vi "UHR-Fleezers Control (host) - 12.7b.vi"() -> ()   [LabVIEW 2012] (continued)
                  tunnel: w664 -> [_ _ _ _ _ _ _ _ _ w685 _ _]
                  tunnel: w663 -> [_ _ _ _ _ _ _ _ _ w683 _ _]
                  frame #0 {
                    n399 = property on="Save ave N" class="DigNum (strict)"("Val(Sgnl)"=1.0 ("Value (Signaling)")) -> ()  [unwired: 2 in, 2 out]
                  }
                  frame #1 {
                    n400 = Wait (ms)(milliseconds to wait=u32 500) -> ()  [unwired: 1 out]
                  }
                  frame #2 {
                    n401 = property on="Trap Delta (MHz)" class="DigNum (strict)"("Val(Sgnl)"="Offset 2 Start (MHz)") -> ()  [unwired: 2 in, 2 out]
                    n402 = Replace Array Subset(array=u32[] [0] ("Index Values"), new element="Offset 2 Set", index=0) -> (w669:u32[])
                    n403 = property on="Saved AOD Raster Scan Parameter Sets" class="Arr (strict)"("Index Values"=w669) -> ()  [unwired: 2 in, 2 out]
                  }
                  frame #3 {
                    n404 = Wait (ms)(milliseconds to wait=u32 500) -> ()  [unwired: 1 out]
                  }
                  frame #4 {
                    n405 = property on="Load parameters" class="Bool (strict)"("Val(Sgnl)"=TRUE ("Value (Signaling)")) -> ()  [unwired: 2 in, 2 out]
                  }
                  frame #5 {
                    n406 = Wait (ms)(milliseconds to wait=u32 500) -> ()  [unwired: 1 out]
                  }
                  frame #6 {
                    n407 = property on="Trap Raster Scan" class="Bool (strict)"("Val(Sgnl)"=TRUE ("Value (Signaling)")) -> ()  [unwired: 2 in, 2 out]
                  }
                  frame #7 {
                    n408 = Wait (ms)(milliseconds to wait=u32 2000) -> ()  [unwired: 1 out]
                  }
                  frame #8 {
                    n409 = while {
                      stop <- w678 stop-if-true
                      n410 = local read "Raster Scanning..."() -> (w681:bool)
                      n411 = local read "Saving..."() -> (w679:bool)
                      n412 = Wait (ms)(milliseconds to wait=u32 100) -> ()  [unwired: 1 out]
                      n413 = Not(x=w679) -> (.not. x?=w677:bool)
                      n414 = Not(x=w681) -> (.not. x?=w680:bool)
                      n415 = And(x=w680, y=w677) -> (x .and. y?=w678:bool)
                    }
                  }
                  frame #9 {
                    n416 = property on="Trap Delta (MHz)" class="DigNum (strict)"("Val(Sgnl)"=w685) -> ()  [unwired: 2 in, 2 out]
                    n417 = property on="Saved AOD Raster Scan Parameter Sets" class="Arr (strict)"("Index Values"=u32[] [0]) -> ()  [unwired: 2 in, 2 out]
                    n418 = property on="Save ave N" class="DigNum (strict)"("Val(Sgnl)"=w683) -> ()  [unwired: 2 in, 2 out]
                  }
                  frame #10 {
                    n419 = Wait (ms)(milliseconds to wait=u32 500) -> ()  [unwired: 1 out]
                  }
                  frame #11 {
                    n420 = property on="Load parameters" class="Bool (strict)"("Val(Sgnl)"=TRUE ("Value (Signaling)")) -> ()  [unwired: 2 in, 2 out]
                  }
                }
              }
            }
          }
          frame #9 {
            n421 = property on="Read Cal" class="Bool (strict)"("Val(Sgnl)"=TRUE ("Value (Signaling)")) -> ()  [unwired: 2 in, 2 out]
          }
          frame #10 {
            n422 = Wait (ms)(milliseconds to wait=u32 1000) -> ()  [unwired: 1 out]
          }
          frame #11 {
            n423 = property on="Fish for Tether" class="Bool (strict)"("Val(Sgnl)"=TRUE ("Value (Signaling)")) -> ()  [unwired: 2 in, 2 out]
          }
        }
        n424 = local write "Cal/Data Acq. Spot"(FALSE ("Cal/Data Acq. Spot")) -> ()
      }
      event "Dump Beads": Value Change {
        n425 = event-data() -> ()  [unwired: 1 in, 5 out]
        n426 = flat-sequence {
          tunnel: ["Dump spot flow on?"] -> w691
          tunnel: [w702] -> w692
          tunnel: w691 -> [w702]
          tunnel: w695 -> [w707]
          tunnel: w694 -> [w706]
          tunnel: [w704] -> w693
          tunnel: w692 -> [w704]
          tunnel: w693 -> [w717]
          frame #0 {
            w696 = FALSE ("Value (Signaling)")
            n427 = local read "Saving..."() -> (w698:bool)
            n428 = local write "Dump Beads"(FALSE ("Dump Beads")) -> ()
            n429 = property on="Inject Pump 3" class="Bool (strict)"("Val(Sgnl)"=w696) -> ()  [unwired: 2 in, 2 out]
            n430 = property on="Inject Pump 1" class="Bool (strict)"("Val(Sgnl)"=w696) -> ()  [unwired: 2 in, 2 out]
            n431 = local write "Stop Saving"(w698) -> ()
          }
          frame #1 {
            w699 = FALSE ("Fl. Triggered...")
            n432 = case shown="True" "Dump spot flow on?" {
              frame False {
              }
              frame True {
                n433 = property on="Sample Channel\nFlow" class="Bool (strict)"("Val(Sgnl)"=TRUE ("Stage Moving")) -> ()  [unwired: 2 in, 2 out]
              }
            }
            n434 = local write "Fl. Triggered..."(w699) -> ()
            n435 = local write "Tether"(w699) -> ()
            n436 = property on="Green Laser ON" class="Bool (strict)"("Val(Sgnl)"=w699) -> ()  [unwired: 2 in, 2 out]
            n437 = property on="Trap Pos. FB ON" class="Bool (strict)"("Val(Sgnl)"=w699) -> ()  [unwired: 2 in, 2 out]
            n438 = property on="Trap Trig. Fl." class="Bool (strict)"("Val(Sgnl)"=w699) -> ()  [unwired: 2 in, 2 out]
            n439 = property on="Fl. Triggered..." class="Bool (strict)"("Val(Sgnl)"=w699) -> ()  [unwired: 2 in, 2 out]
            n440 = property on="Dip for Protein" class="Bool (strict)"("Val(Sgnl)"=w699) -> ()  [unwired: 2 in, 2 out]
            n441 = property on="Pause dwell" class="Bool (strict)"("Val(Sgnl)"=w699) -> ()  [unwired: 2 in, 2 out]
          }
          frame #2 {
            n442 = property on="Trap Pos. FB Offset Factor" class="DigNum (strict)"("Val(Sgnl)"=i64 0 ("Value (Signaling)")) -> ()  [unwired: 2 in, 2 out]
          }
          frame #3 {
            n443 = local read "Saved Stage Positions"() -> (w708:dbl[][])
            n444 = local write "Stage Moving"(TRUE ("Stage Moving")) -> ()
            n445 = Array Subset(array=w708, index (row)=3 ("index"), length (row)=1 ("length"), index (col)=1 ("index"), length (col)=3 ("length")) -> (w713:dbl[][])
            n446 = Reshape Array(w713, 3 ("dimension size")) -> (w711:dbl[])
            n447 = Array To Cluster(array=w711) -> (cluster=w710:cluster{"[0]":dbl, "[1]":dbl, "[2]":dbl})
            n448 = call "Set Stage Position.vi"("Position"=w710, "error in"=w706, "VISA resource name in"=w707) -> ()  [unwired: 3 out]
          }
          frame #4 {
            w718 = FALSE ("Value (Signaling)")
            n449 = case shown="True" w717 {
              frame False {
              }
              frame True {
                n450 = property on="Sample Channel\nFlow" class="Bool (strict)"("Val(Sgnl)"=FALSE ("Stage Moving")) -> ()  [unwired: 2 in, 2 out]
              }
            }
            n451 = property on="Trap 1 (ON/OFF)" class="Bool (strict)"("Val(Sgnl)"=w718) -> ()  [unwired: 2 in, 2 out]
            n452 = property on="Trap 2 (ON/OFF)" class="Bool (strict)"("Val(Sgnl)"=w718) -> ()  [unwired: 2 in, 2 out]
            n453 = call <vilib>:"Beep.vi"() -> ()  [unwired: 3 in, 9 out]
          }
          frame #5 {
            n454 = property on="Move Cap. 2 (ADig Top)" class="Bool (strict)"("Val(Sgnl)"=TRUE ("Value (Signaling)")) -> ()  [unwired: 2 in, 2 out]
            n455 = property on="Tab Control" class="TabCtl (strict)"("Val(Sgnl)"=T26."Status" ("Value (Signaling)")) -> ()  [unwired: 2 in, 2 out]
          }
        }
      }
      event "Dip for Protein": Value Change {
        n456 = event-data() -> ()  [unwired: 1 in, 5 out]
        n457 = case shown="True" "Dip for Protein" {
          tunnel: w724 -> [_ w726]
          tunnel: w723 -> [_ w725]
          frame False {
          }
          frame True {
            n458 = while {
              tunnel: w726 -> [w737]
              tunnel: w725 -> [w736]
              i -> [w731]
              stop <- w733 stop-if-true
              n459 = Increment(x=w731) -> (x+1=→"Dip #":i32)
              n460 = flat-sequence {
                tunnel: w736 -> [w748]
                tunnel: w737 -> [w749]
                tunnel: [w749] -> w741
                tunnel: [w748] -> w740
                tunnel: [w742] -> w727
                tunnel: [w754] -> w735
                tunnel: [w755] -> w734
                tunnel: w741 -> [w756]
                tunnel: w740 -> [w757]
                tunnel: [w752] -> w728
                tunnel: w727 -> [w752]
                tunnel: [w765] -> w739
                tunnel: w735 -> [w765]
                tunnel: [w764] -> w738
                tunnel: w734 -> [w764]
                tunnel: [w761] -> w732
                tunnel: [w760] -> w729
                tunnel: w728 -> [w760]
                tunnel: w738 -> [w785]
                tunnel: w739 -> [w786]
                tunnel: w732 -> [w787]
                tunnel: w729 -> [w784]
                tunnel: [w843] -> w733
                frame #0 {
                  n461 = local read "Trap Pos. FB ON"() -> (w742:bool)
                  n462 = Compound Arithmetic op=AND("Flow ON\nduring dip?", "FB OFF when \nflow ON", w742) -> (w743:bool)
                  n463 = case shown="True" "Move trap \nbefore dip move?" {
                    frame False {
                    }
                    frame True {
                      n464 = property on="Trap Delta (MHz)" class="DigNum (strict)"("Val(Sgnl)"="Dipping Delta (MHz)") -> ()  [unwired: 2 in, 2 out]
                    }
                  }
                  n465 = property on="Green Laser ON" class="Bool (strict)"("Val(Sgnl)"="Green ON\nbefore dip?") -> ()  [unwired: 2 in, 2 out]
                  n466 = property on="Sample Channel\nFlow" class="Bool (strict)"("Val(Sgnl)"="Flow ON\nduring dip?") -> ()  [unwired: 2 in, 2 out]
                  n467 = case shown="True" w743 {
                    frame False {
                    }
                    frame True {
                      n468 = property on="Trap Pos. FB ON" class="Bool (strict)"("Val(Sgnl)"=FALSE ("Value (Signaling)")) -> ()  [unwired: 2 in, 2 out]
                    }
                  }
                }
                frame #1 {
                  n469 = local read "Saved Stage Positions"() -> (w759:dbl[][])
                  n470 = local write "Cancel dwell"(FALSE ("Cancel dwell")) -> ()
                  n471 = call "move to saved stage position.vi"("error in"=w757, "Stage VISA resource name in"=w756, "Position"="Dip Stage \nPosition", "Saved Stage Positions"=w759) -> ("VISA resource name out"=w754:refnum<visa-resource-name>, "error out"=w755:errorcluster)
                }
                frame #2 {
                  n472 = node-c288() -> (w763:T23)  [unwired: 4 in]
                  n473 = timed-loop {
                    timing: w763 -> [_]
                    timing-out: [_] -> w762
                    tunnel: [w769] -> w761
                    i -> [w766]
                    stop <- w770 stop-if-true
                    n474 = node-c288() -> ()  [unwired: 1 in, 1 out]
                    n475 = Greater Or Equal?(x=w766, y="Dip Duration (s)") -> (x >= y?=w778:bool)
                    n476 = local read "Dip for Protein"() -> (w771:bool)
                    n477 = local read "Dump Beads"() -> (w768:bool)
                    n478 = local read "Cancel dwell"() -> (w777:bool)
                    n479 = local read "Pause dwell"() -> (w774:bool)
                    n480 = Not(x=w771) -> (.not. x?=w776:bool)
                    n481 = Compound Arithmetic op=OR(w777, w778, w776) -> (w775:bool)
                    n482 = Select(t=FALSE, s=w774, f=w775) -> (s? t:f=w772:bool)
                    n483 = Not(x=w768) -> (.not. x?=w767:bool)
                    n484 = node-c288() -> ()  [unwired: 1 in, 1 out]
                    n485 = And(x=w771, y=w767) -> (x .and. y?=w769:bool)
                    n486 = Or(x=w772, y=w768) -> (x .or. y?=w770:bool)
                    "Dip Time (s)" <- w766
                  }
                  n487 = node-c288(w762) -> ()  [unwired: 1 out]
                }
                frame #3 {
                  n488 = case shown="True" w787 {
                    tunnel: w786 -> [_ w792]
                    tunnel: w785 -> [_ w791]
                    tunnel: w784 -> [_ w788]
                    frame False {
                    }
                    frame True {
                      n489 = flat-sequence {
                        tunnel: w791 -> [w796]
                        tunnel: w792 -> [w797]
                        tunnel: [w797] -> w790
                        tunnel: [w796] -> w789
                        tunnel: w788 -> [w793]
                        tunnel: w790 -> [w807]
                        tunnel: w789 -> [w806]
                        tunnel: w788 -> [w815]
                        frame #0 {
                          n490 = local read "Sample Channel\nFlow"() -> (w795:bool)
                          n491 = case shown="True" w795 {
                            tunnel: "Flow ON \nduring return\nfrom dip?" -> [w798 w801]
                            tunnel: w793 -> [_ w800]
                            frame False {
                              n492 = case shown="True" w798 {
                                frame False {
                                }
                                frame True {
                                n493 = property on="Sample Channel\nFlow" class="Bool (strict)"("Val(Sgnl)"=TRUE ("Value (Signaling)")) -> ()  [unwired: 2 in, 2 out]
                                }
                              }
                            }
                            frame True {
                              n494 = case shown="False" w801 {
                                tunnel: w800 -> [w802 _]
                                frame False {
                                n495 = property on="Trap Pos. FB ON" class="Bool (strict)"("Val(Sgnl)"=w802) -> ()  [unwired: 2 in, 2 out]
                                n496 = property on="Sample Channel\nFlow" class="Bool (strict)"("Val(Sgnl)"=FALSE ("Value (Signaling)")) -> ()  [unwired: 2 in, 2 out]
                                }
                                frame True {
                                }
                              }
                            }
                          }
                        }
                        frame #1 {
                          # "For turning on green laser before stage reaches lower spot"
                          n497 = case shown="True" "Green ON\nafter start\nreturn?" {
                            frame False {
                            }
                            frame True {
                              n498 = flat-sequence {
                                frame #0 {
                                n499 = Multiply(x="Green delay after \nstart return (s)", y=1000.0) -> (x*y=w812:dbl)
                                n500 = Wait (ms)(milliseconds to wait=w812) -> ()  [unwired: 1 out]
                                }
                                frame #1 {
                                n501 = property on="Green Laser ON" class="Bool (strict)"("Val(Sgnl)"=TRUE ("Value (Signaling)")) -> ()  [unwired: 2 in, 2 out]
                                }
                              }
                            }
                          }
                          n502 = local read "Saved Stage Positions"() -> (w810:dbl[][])
                          n503 = local write "Cancel dwell"(FALSE ("Cancel dwell")) -> ()
                          n504 = call "move to saved stage position.vi"("error in"=w806, "Stage VISA resource name in"=w807, "Position"="Return Stage \nPosition", "Saved Stage Positions"=w810) -> ("error out"=w808:errorcluster)  [unwired: 1 out]
                          n505 = local write "Stage Control Serial Error"(w808) -> ()
                        }
                        frame #2 {
                          n506 = property on="Trap Pos. FB ON" class="Bool (strict)"("Val(Sgnl)"=w815) -> ()  [unwired: 2 in, 2 out]
                          n507 = case shown="True" "Green ON \nafter return?" {
                            frame False {
                            }
                            frame True {
                              n508 = property on="Green Laser ON" class="Bool (strict)"("Val(Sgnl)"=TRUE ("Value (Signaling)")) -> ()  [unwired: 2 in, 2 out]
                            }
                          }
                          n509 = case shown="True" "Move trap after return?" {
                            frame False {
                            }
                            frame True {
                              n510 = property on="Trap Delta (MHz)" class="DigNum (strict)"("Val(Sgnl)"="Dip Trap Delta 2 (MHz)") -> ()  [unwired: 2 in, 2 out]
                            }
                          }
                          n511 = case shown="True" "Save data after return?" {
                            frame False {
                            }
                            frame True {
                              n512 = property on="Start Saving" class="Bool (strict)"("Val(Sgnl)"=TRUE ("Value (Signaling)")) -> ()  [unwired: 2 in, 2 out]
                            }
                          }
                          n513 = property on="Sample Channel\nFlow" class="Bool (strict)"("Val(Sgnl)"="Flow ON\nduring daq?") -> ()  [unwired: 2 in, 2 out]
                        }
                        frame #3 {
                          n514 = node-c288() -> (w824:T23)  [unwired: 4 in]
                          n515 = timed-loop {
                            timing: w824 -> [_]
                            timing-out: [_] -> w823
                            i -> [w825]
                            stop <- w827 stop-if-true
                            n516 = node-c288() -> ()  [unwired: 1 in, 1 out]
                            n517 = local read "Dump Beads"() -> (w826:bool)
                            n518 = Greater Or Equal?(x=w825, y="Dwell Duration (s)") -> (x >= y?=w832:bool)
                            n519 = local read "Dip for Protein"() -> (w829:bool)
                            n520 = Not(x=w829) -> (.not. x?=w828:bool)
                            n521 = Compound Arithmetic op=OR(w832, "Cancel dwell", w828) -> (w831:bool)
                            n522 = node-c288() -> ()  [unwired: 1 in, 1 out]
                            n523 = Select(t=FALSE, s="Pause dwell", f=w831) -> (s? t:f=w834:bool)
                            n524 = Or(x=w834, y=w826) -> (x .or. y?=w827:bool)
                            "Dwell Time (s)" <- w825
                          }
                          n525 = node-c288(w823) -> ()  [unwired: 1 out]
                        }
                      }
                    }
                  }
                }
                frame #4 {
                  n526 = local read "Dip for Protein"() -> (w844:bool)
                  n527 = local read "Dump Beads"() -> (w841:bool)
                  n528 = local write "Cancel dwell"(FALSE ("Cancel dwell")) -> ()
                  n529 = Not(x=w844) -> (.not. x?=w845:bool)
                  n530 = Not(x="Cont. Repeat Dipping?") -> (.not. x?=w847:bool)
                  n531 = Compound Arithmetic op=OR(w845, w847, w841) -> (w843:bool)
                }
              }
            }
          }
        }
      }
      event "Profile": Value Change {
        n532 = event-data() -> ()  [unwired: 1 in, 5 out]
        n533 = flat-sequence {
          tunnel: w856 -> [w859]
          tunnel: w855 -> [w867]
          tunnel: [w861] -> w854
          tunnel: [w860] -> w853
          tunnel: [w858] -> w851
          tunnel: [w857] -> w848
          tunnel: w854 -> [w874]
          tunnel: w853 -> [w873]
          tunnel: [w871] -> w852
          tunnel: w851 -> [w872]
          tunnel: [w870] -> w850
          tunnel: [w869] -> w849
          tunnel: w848 -> [w869]
          tunnel: w852 -> [w878]
          tunnel: w850 -> [w877]
          tunnel: w849 -> [w876]
          frame #0 {
            n534 = call "Read Stage Position.vi"("error in"=w867, "VISA resource name in"=w859) -> ("Current Position"=w857:cluster{dbl, dbl, dbl}, "error out"=w860:errorcluster, "VISA resource name out"=w858:refnum<visa-resource-name>)  [unwired: 1 out]
            "Current Position" <- w857
            n535 = local write "Stage Control Serial Error"(w860) -> ()
            n536 = Unbundle(w857) -> (w864:dbl, w866:dbl, w862:dbl)
            n537 = Add(x=w866, y="Y change (mm)") -> (x+y=w863:dbl)
            n538 = Bundle(w864, w863, w862) -> (w861:cluster{dbl, dbl, dbl})  [unwired: 1 in]
          }
          frame #1 {
            # "move to new position and start saving"
            n539 = local write "Stage Moving"(TRUE ("Stage Moving")) -> ()
            n540 = local write "Start Saving"(TRUE ("Start Saving")) -> ()
            n541 = call "Set Stage Position.vi"("Position"=w874, "error in"=w873, "VISA resource name in"=w872) -> ("error out"=w870:errorcluster, "VISA resource name out"=w871:refnum<visa-resource-name>)  [unwired: 1 out]
          }
          frame #2 {
            # "go back to start"
            n542 = call "Set Stage Position.vi"("Position"=w876, "error in"=w877, "VISA resource name in"=w878) -> ()  [unwired: 3 out]
          }
          frame #3 {
            # "stop saving"
            n543 = local write "Stop Saving"(TRUE ("Stop Saving")) -> ()
            n544 = local write "Stage Moving"(FALSE ("Stage Moving")) -> ()
          }
        }
      }
      event "Move to Position 1", "Move to Position 2", "Move to Position 3", "Move to Position 4", "Move to Position 5", "Lower Ch. Cap.": Value Change {
        n545 = event-data() -> ()  [unwired: 1 in, 5 out]
        n546 = Or(x="Move to Position 5", y="Lower Ch. Cap.") -> (x .or. y?=w884:bool)
        n547 = Build Array("Move to Position 1", "Move to Position 2", "Move to Position 3", "Move to Position 4", w884) -> (w887:bool[])
        n548 = Boolean Array To Number(Boolean array=w887) -> (number=w886:u32)
        n549 = Logarithm Base 2(1:w886) -> (0:w885:dbl)
        n550 = flat-sequence {
          tunnel: w885 -> [w896]
          tunnel: w882 -> [w894]
          tunnel: w881 -> [w893]
          frame #0 {
            n551 = local read "Saved Stage Positions"() -> (w904:dbl[][])
            n552 = Array Subset(array=w904, index (row)=w896, length (row)=1 ("length"), index (col)=1 ("index"), length (col)=3 ("length")) -> (w901:dbl[][])
            n553 = Reshape Array(w901, 3 ("dimension size")) -> (w899:dbl[])
            n554 = Array To Cluster(array=w899) -> (cluster=w898:cluster{"[0]":dbl, "[1]":dbl, "[2]":dbl})
            n555 = call "Set Stage Position.vi"("Position"=w898, "error in"=w893, "VISA resource name in"=w894) -> ("error out"=w897:errorcluster)  [unwired: 2 out]
            n556 = local write "Stage Moving"(TRUE ("Stage Moving")) -> ()
            n557 = local write "Stage Control Serial Error"(w897) -> ()
          }
          frame #1 {
            n558 = local write "Stage Moving"(FALSE ("Stage Moving")) -> ()
            n559 = call <vilib>:"Beep.vi"() -> ()  [unwired: 3 in, 9 out]
          }
        }
      }
      event "Got ADig bead": Value Change {
        n560 = event-data() -> ()  [unwired: 1 in, 5 out]
        n561 = flat-sequence {
          frame #0 {
            n562 = local read "Cap 1 Samp Flow ON"() -> (w908:bool)
            n563 = case shown="True" w908 {
              frame False {
              }
              frame True {
                n564 = property on="Sample Channel\nFlow" class="Bool (strict)"("Val(Sgnl)"=TRUE ("Value (Signaling)")) -> ()  [unwired: 2 in, 2 out]
              }
            }
          }
          frame #1 {
            n565 = property on="Inject Pump 3" class="Bool (strict)"("Val(Sgnl)"=FALSE ("Value (Signaling)")) -> ()  [unwired: 2 in, 2 out]
          }
          frame #2 {
            n566 = property on="Move Cap. 1 (DNA Bottom)" class="Bool (strict)"("Val(Sgnl)"=TRUE ("Value (Signaling)")) -> ()  [unwired: 2 in, 2 out]
          }
        }
      }
      event "Force FB Data\nScript": Value Change {
        n567 = event-data() -> ()  [unwired: 1 in, 5 out]
        n568 = flat-sequence {
          tunnel: w917 -> [w921]
          tunnel: w918 -> [w922]
          tunnel: [w922] -> w913
          tunnel: [w921] -> w912
          tunnel: w913 -> [w925]
          tunnel: w912 -> [w924]
          tunnel: ["Trap Trig Fl."] -> w914
          tunnel: [w950] -> w915
          tunnel: w914 -> [w950]
          tunnel: [w954] -> w916
          tunnel: w915 -> [w954]
          tunnel: w916 -> [w956]
          frame #0 {
            n569 = property on="Trap Delta (MHz)" class="DigNum (strict)"("Val(Sgnl)"="Trap Delta Before Moving") -> ()  [unwired: 2 in, 2 out]
          }
          frame #1 {
            n570 = local read "Saved Stage Positions"() -> (w927:dbl[][])
            n571 = local write "FB Trap Pos Offset"(0.0 ("FB Trap Pos Offset")) -> ()
            n572 = property on="Trap Pos. FB Offset Factor" class="DigNum (strict)"("Val(Sgnl)"=i64 0 ("Value (Signaling)")) -> ()  [unwired: 2 in, 2 out]
            n573 = local write "Stage Moving"(TRUE ("Stage Moving")) -> ()
            n574 = call "move to saved stage position.vi"("error in"=w924, "Stage VISA resource name in"=w925, "Position"="Stage Position To Establish FB", "Saved Stage Positions"=w927) -> ("error out"=w923:errorcluster)  [unwired: 1 out]
            n575 = local write "Stage Control Serial Error"(w923) -> ()
          }
          frame #2 {
            n576 = call <vilib>:"Beep.vi"() -> ()  [unwired: 3 in, 9 out]
            n577 = Multiply(x="Wait (s)", y=u32 1000 ("milliseconds to wait")) -> (x*y=w934:u32)
            n578 = property on="Trap Delta (MHz)" class="DigNum (strict)"("Val(Sgnl)"="Starting \nTrap Delta (MHz)") -> ()  [unwired: 2 in, 2 out]
            n579 = local write "Stage Moving"(FALSE ("Stage Moving")) -> ()
            n580 = Wait (ms)(milliseconds to wait=w934) -> ()  [unwired: 1 out]
            n581 = property on="Tab Control 2" class="TabCtl (strict)"("Val(Sgnl)"=T6."Feedback on Trap Position" ("Value (Signaling)")) -> ()  [unwired: 2 in, 2 out]
            n582 = property on="Tab Control" class="TabCtl (strict)"("Val(Sgnl)"=T27."Trap Control (RF)" ("Value (Signaling)")) -> ()  [unwired: 2 in, 2 out]
          }
          frame #3 {
            n583 = property on="Set Reading to\nSetpoint" class="Bool (strict)"("Val(Sgnl)"=TRUE ("Value (Signaling)")) -> ()  [unwired: 2 in, 2 out]
            n584 = Wait (ms)(milliseconds to wait=u32 500) -> ()  [unwired: 1 out]
          }
          frame #4 {
            n585 = property on="Trap Pos. FB ON" class="Bool (strict)"("Val(Sgnl)"=TRUE ("Value (Signaling)")) -> ()  [unwired: 2 in, 2 out]
            n586 = Wait (ms)(milliseconds to wait=u32 250) -> ()  [unwired: 1 out]
          }
          frame #5 {
            n587 = case shown="False" "Trap Trig Fl." {
              frame False {
                n588 = case shown="True" "Green ON after FB ON?" {
                  selector: "Green ON after FB ON?" -> [_ w949]
                  frame False {
                  }
                  frame True {
                    n589 = property on="Green Laser ON" class="Bool (strict)"("Val(Sgnl)"=w949) -> ()  [unwired: 2 in, 2 out]
                  }
                }
              }
              frame True {
              }
            }
            n590 = case shown="True" "Remove Action Offset" {
              tunnel: TRUE ("Value (Signaling)") -> [w946 w947]
              frame False {
                n591 = property on="Remove Unwinding Offset" class="Bool (strict)"("Val(Sgnl)"=w946) -> ()  [unwired: 2 in, 2 out]
              }
              frame True {
                n592 = property on="Remove Action Offset" class="Bool (strict)"("Val(Sgnl)"=w947) -> ()  [unwired: 2 in, 2 out]
              }
            }
            n593 = Wait (ms)(milliseconds to wait=u32 250) -> ()  [unwired: 1 out]
          }
          frame #6 {
            n594 = property on="Start Saving" class="Bool (strict)"("Val(Sgnl)"=TRUE ("Value (Signaling)")) -> ()  [unwired: 2 in, 2 out]
            n595 = Wait (ms)(milliseconds to wait=u32 5000) -> ()  [unwired: 1 out]
          }
          frame #7 {
            w953 = TRUE ("Value (Signaling)")
            n596 = property on="Rem fb disp offset" class="Bool (strict)"("Val(Sgnl)"=w953) -> ()  [unwired: 2 in, 2 out]
            n597 = property on="Remove Offset" class="Bool (strict)"("Val(Sgnl)"=w953) -> ()  [unwired: 2 in, 2 out]
            n598 = Wait (ms)(milliseconds to wait=u32 100) -> ()  [unwired: 1 out]
          }
          frame #8 {
            n599 = case shown="True" w956 {
              frame False {
              }
              frame True {
                n600 = local write "Trap Trig. Fl."(TRUE ("Value (Signaling)")) -> ()
              }
            }
          }
          frame #9 {
            n601 = case shown="True" "Start dipping after?" {
              frame False {
              }
              frame True {
                n602 = flat-sequence {
                  frame #0 {
                    n603 = Multiply(x="Delay before dipping (s)", y=1000.0) -> (x*y=w960:dbl)
                    n604 = Wait (ms)(milliseconds to wait=w960) -> ()  [unwired: 1 out]
                  }
                  frame #1 {
                    n605 = property on="Dip for Protein" class="Bool (strict)"("Val(Sgnl)"=TRUE ("Value (Signaling)")) -> ()  [unwired: 2 in, 2 out]
                    n606 = local write "Scripts"(T1."Dipping" ("Scripts")) -> ()
                  }
                }
              }
            }
          }
        }
      }
      event "Fixed Traps Data\nScript": Value Change {
        n607 = event-data() -> ()  [unwired: 1 in, 5 out]
        n608 = flat-sequence {
          frame #0 {
            n609 = case shown="True" "Green ON" {
              frame False {
              }
              frame True {
                n610 = property on="Green Laser ON" class="Bool (strict)"("Val(Sgnl)"=TRUE) -> ()  [unwired: 2 in, 2 out]
              }
            }
            n611 = local write "Offset (nm)"(0.0 ("Offset (nm)")) -> ()
            n612 = property on="Sample Channel\nFlow" class="Bool (strict)"("Val(Sgnl)"=FALSE ("Value (Signaling)")) -> ()  [unwired: 2 in, 2 out]
            n613 = property on="Trap Delta (MHz)" class="DigNum (strict)"("Val(Sgnl)"="Fixed Traps Trap Delta (MHz)") -> ()  [unwired: 2 in, 2 out]
          }
          frame #1 {
            n614 = Wait (ms)(milliseconds to wait=u32 1000) -> ()  [unwired: 1 out]
          }
          frame #2 {
            n615 = local write "Start Saving"(TRUE ("Start Saving")) -> ()
          }
          frame #3 {
            n616 = local read "Bead Sep. Int. Time (s)"() -> (w971:dbl)
            n617 = Multiply(x=w971, y=1000.0) -> (x*y=w973:dbl)
            n618 = Wait (ms)(milliseconds to wait=w973) -> ()  [unwired: 1 out]
          }
          frame #4 {
            n619 = property on="Remove Offset" class="Bool (strict)"("Val(Sgnl)"=TRUE ("Value (Signaling)")) -> ()  [unwired: 2 in, 2 out]
          }
          frame #5 {
            n620 = property on="Dip for Protein" class="Bool (strict)"("Val(Sgnl)"="Start dipping after?") -> ()  [unwired: 2 in, 2 out]
          }
        }
      }
      event "Got DNA bead": Value Change {
        n621 = event-data() -> ()  [unwired: 1 in, 5 out]
        n622 = flat-sequence {
          frame #0 {
            n623 = local read "Daq spot flow on"() -> (w978:bool)
            n624 = case shown="True" w978 {
              frame False {
              }
              frame True {
                n625 = property on="Sample Channel\nFlow" class="Bool (strict)"("Val(Sgnl)"=TRUE ("Value (Signaling)")) -> ()  [unwired: 2 in, 2 out]
              }
            }
            n626 = property on="Got DNA bead" class="Bool"("Key Focus"=FALSE) -> ()  [unwired: 2 in, 2 out]
          }
          frame #1 {
            n627 = property on="Inject Pump 1" class="Bool (strict)"("Val(Sgnl)"=FALSE ("Value (Signaling)")) -> ()  [unwired: 2 in, 2 out]
          }
          frame #2 {
            n628 = property on="Cal/Data Acq. Spot" class="Bool (strict)"("Val(Sgnl)"=TRUE ("Value (Signaling)")) -> ()  [unwired: 2 in, 2 out]
          }
        }
      }
      event "Take Stepping Data": Value Change {
        n629 = event-data() -> ()  [unwired: 1 in, 5 out]
        n630 = local read "Save ave N"() -> (w990:dbl)
        n631 = flat-sequence {
          tunnel: w990 -> [w992]
          tunnel: [w992] -> w985
          tunnel: [w994] -> w986
          tunnel: w985 -> [w994]
          tunnel: [w996] -> w987
          tunnel: w986 -> [w996]
          tunnel: [w999] -> w988
          tunnel: w987 -> [w999]
          tunnel: [w1001] -> w989
          tunnel: w988 -> [w1001]
          tunnel: [w1003] -> w983
          tunnel: w989 -> [w1003]
          tunnel: w983 -> [w1006]
          tunnel: [w1006] -> w982
          tunnel: w982 -> [w1007]
          tunnel: [w1007] -> w984
          tunnel: w984 -> [w1013]
          frame #0 {
            n632 = property on="Save ave N" class="DigNum (strict)"("Val(Sgnl)"="Save ave factor") -> ()  [unwired: 2 in, 2 out]
          }
          frame #1 {
            n633 = Wait (ms)(milliseconds to wait=u32 100) -> ()  [unwired: 1 out]
          }
          frame #2 {
            n634 = local read "Offset 2 Start (MHz)"() -> (w998:dbl)
            n635 = property on="Saved AOD Raster Scan Parameter Sets" class="Arr (strict)"("Index Values"=u32[] [2]) -> ()  [unwired: 2 in, 2 out]
            n636 = property on="Trap Delta (MHz)" class="DigNum (strict)"("Val(Sgnl)"=w998) -> ()  [unwired: 2 in, 2 out]
          }
          frame #3 {
            n637 = property on="Load parameters" class="Bool (strict)"("Val(Sgnl)"=TRUE ("Value (Signaling)")) -> ()  [unwired: 2 in, 2 out]
          }
          frame #4 {
            n638 = Wait (ms)(milliseconds to wait=u32 100) -> ()  [unwired: 1 out]
          }
          frame #5 {
            n639 = property on="Trap Raster Scan" class="Bool (strict)"("Val(Sgnl)"=TRUE ("Value (Signaling)")) -> ()  [unwired: 2 in, 2 out]
          }
          frame #6 {
            n640 = Wait (ms)(milliseconds to wait=u32 1000) -> ()  [unwired: 1 out]
          }
          frame #7 {
            n641 = while {
              stop <- w1010 stop-if-true
              n642 = local read "Raster Scanning..."() -> (w1012:bool)
              n643 = local read "Saving..."() -> (w1011:bool)
              n644 = Not(x=w1011) -> (.not. x?=w1008:bool)
              n645 = Not(x=w1012) -> (.not. x?=w1009:bool)
              n646 = And(x=w1009, y=w1008) -> (x .and. y?=w1010:bool)
            }
          }
          frame #8 {
            n647 = property on="Save ave N" class="DigNum (strict)"("Val(Sgnl)"=w1013) -> ()  [unwired: 2 in, 2 out]
          }
        }
      }
      event "Step Size (nm)": Value Change {
        n648 = event-data() -> ()  [unwired: 1 in, 5 out]
        n649 = flat-sequence {
          frame #0 {
            n650 = property on="Saved AOD Raster Scan Parameter Sets" class="Arr (strict)"("Index Values"=u32[] [1]) -> ()  [unwired: 2 in, 2 out]
          }
          frame #1 {
            n651 = Multiply(x="N Steps", y="Step Size (nm)") -> (x*y=w1015:dbl)
            n652 = property on="Scan Speed AOD (nm/s) 2" class="DigNum (strict)"("Value"="Step Size (nm)") -> ()  [unwired: 2 in, 2 out]
            n653 = property on="Step Size AOD (nm) 2" class="DigNum (strict)"("Value"="Step Size (nm)") -> ()  [unwired: 2 in, 2 out]
            n654 = property on="Scan Range AOD (nm) 2" class="DigNum (strict)"("Value"=w1015) -> ()  [unwired: 2 in, 2 out]
          }
        }
      }
      event "Take Detection Laser\nImage": Value Change {
        n655 = event-data() -> ()  [unwired: 1 in, 5 out]
        n656 = flat-sequence {
          tunnel: [w1043] -> w1033
          tunnel: [w1042] -> w1026
          tunnel: [w1041] -> w1018
          tunnel: [w1046] -> w1034
          tunnel: w1033 -> [w1046]
          tunnel: [w1045] -> w1027
          tunnel: w1026 -> [w1045]
          tunnel: [w1044] -> w1019
          tunnel: w1018 -> [w1044]
          tunnel: [w1050] -> w1035
          tunnel: w1034 -> [w1050]
          tunnel: [w1049] -> w1028
          tunnel: w1027 -> [w1049]
          tunnel: [w1048] -> w1020
          tunnel: w1019 -> [w1048]
          tunnel: [w1056] -> w1036
          tunnel: w1035 -> [w1056]
          tunnel: [w1055] -> w1029
          tunnel: w1028 -> [w1055]
          tunnel: [w1054] -> w1021
          tunnel: w1020 -> [w1054]
          tunnel: [w1060] -> w1037
          tunnel: w1036 -> [w1060]
          tunnel: [w1059] -> w1030
          tunnel: w1029 -> [w1059]
          tunnel: [w1058] -> w1022
          tunnel: w1021 -> [w1058]
          tunnel: [w1064] -> w1038
          tunnel: w1037 -> [w1064]
          tunnel: [w1063] -> w1031
          tunnel: w1030 -> [w1063]
          tunnel: [w1062] -> w1023
          tunnel: w1022 -> [w1062]
          tunnel: [w1068] -> w1039
          tunnel: w1038 -> [w1068]
          tunnel: [w1067] -> w1032
          tunnel: w1031 -> [w1067]
          tunnel: [w1066] -> w1024
          tunnel: w1023 -> [w1066]
          tunnel: w1039 -> [w1074]
          tunnel: w1032 -> [w1073]
          tunnel: [w1071] -> w1025
          tunnel: w1024 -> [w1071]
          tunnel: w1025 -> [w1075]
          frame #0 {
            n657 = local read "Laser interlacing mode"() -> (w1042:enum32{"Laser ON", "Laser OFF", "Interlace"})
            n658 = local read "Green FB On/Off"() -> (w1041:bool)
            n659 = local read "Green Laser ON"() -> (w1043:bool)
          }
          frame #1 {
            n660 = property on="Green FB On/Off" class="Bool (strict)"("Val(Sgnl)"=FALSE ("Value (Signaling)")) -> ()  [unwired: 2 in, 2 out]
          }
          frame #2 {
            n661 = property on="Green Laser ON" class="Bool (strict)"("Val(Sgnl)"=TRUE ("Value (Signaling)")) -> ()  [unwired: 2 in, 2 out]
            n662 = property on="Flip Green Filter" class="Bool (strict)"("Val(Sgnl)"=TRUE ("Value (Signaling)")) -> ()  [unwired: 2 in, 2 out]
            n663 = property on="Laser interlacing mode" class="RadioBtnsControl (strict)"("Val(Sgnl)"=enum32{"Laser ON", "Laser OFF", "Interlace"}."Laser ON" ("Value (Signaling)")) -> ()  [unwired: 2 in, 2 out]
          }
          frame #3 {
            n664 = Wait (ms)(milliseconds to wait=u32 500) -> ()  [unwired: 1 out]
          }
          frame #4 {
            n665 = property on="Confocal Image" class="Bool (strict)"("Val(Sgnl)"=TRUE ("Value (Signaling)")) -> ()  [unwired: 2 in, 2 out]
          }
          frame #5 {
            n666 = Wait (ms)(milliseconds to wait=u32 2000) -> ()  [unwired: 1 out]
          }
          frame #6 {
            n667 = while {
              stop <- w1069 stop-if-true
              n668 = local read "Saving..."() -> (w1070:bool)
              n669 = Not(x=w1070) -> (.not. x?=w1069:bool)
            }
          }
          frame #7 {
            n670 = property on="Flip Green Filter" class="Bool (strict)"("Val(Sgnl)"=TRUE ("Value (Signaling)")) -> ()  [unwired: 2 in, 2 out]
            n671 = property on="Green Laser ON" class="Bool (strict)"("Val(Sgnl)"=w1074) -> ()  [unwired: 2 in, 2 out]
            n672 = property on="Laser interlacing mode" class="RadioBtnsControl (strict)"("Val(Sgnl)"=w1073) -> ()  [unwired: 2 in, 2 out]
          }
          frame #8 {
            n673 = property on="Green FB On/Off" class="Bool (strict)"("Val(Sgnl)"=w1075) -> ()  [unwired: 2 in, 2 out]
          }
        }
      }
      event "Move in a Circle": Value Change {
        # "converting distance (d) to angle (a)\na=arcsin(d/2r)"
        # "radius"
        # "radius"
        # "T1 Y"
        # "T1 X"
        n674 = event-data() -> ()  [unwired: 1 in, 5 out]
        n675 = local read "BD 2 Frequency 1 (MHz)"() -> (w1080:dbl)
        n676 = local read "BD 1 Frequency 2 (MHz)"() -> (w1079:dbl)
        n677 = local read "BD 2 Frequency 2 (MHz)"() -> (w1078:dbl)
        n678 = local read "BD 1 Frequency 1 (MHz)"() -> (w1081:dbl)
        n679 = Subtract(x=w1080, y="Center Y Frequency (MHz)") -> (x-y=w1090:dbl)
        n680 = Absolute Value(x=w1090) -> (abs(x)=w1086:dbl)
        n681 = Multiply(x=w1086, y=2) -> (x*y=w1085:dbl)
        n682 = Divide(x="2D Motion Trap Separation (MHz)", y=w1085) -> (x/y=w1083:dbl)
        n683 = Inverse Sine(1:w1083) -> (0:w1087:dbl)
        n684 = Multiply(x=w1087, y=2) -> (x*y=w1082:dbl)
        n685 = node-c288() -> (w1092:T23)  [unwired: 4 in]
        n686 = timed-loop {
          tunnel: w1086 -> [w1119]
          timing: w1092 -> [_]
          timing-out: [_] -> w1091
          tunnel: w1081 -> [w1110]
          tunnel: w1080 -> [w1109]
          tunnel: w1082 -> [w1117]
          tunnel: w1079 -> [w1115]
          tunnel: w1078 -> [_]
          tunnel: "Center Y Frequency (MHz)" -> [w1114]
          shift-right: [w1095] -> _
          shift-left: dbl[] [] -> [w1098]
          shift-right: [w1094] -> _
          shift-left: _ -> [w1096]
          i -> [w1127]
          stop <- w1107 stop-if-true
          # "r"
          # "r"
          # "r"
          # "r"
          # "\"omega*t\""
          # "Trap 2"
          # "Trap separation (radians)"
          # "Trap 1"
          # "Offset (starts\n at bottom of\n the circle)"
          # "\"t\""
          # "\"omega\""
          n687 = node-c288() -> (w1129:i64)  [unwired: 1 in]
          n688 = Divide(x=w1129, y=1000) -> (x/y=w1128:dbl)
          n689 = Multiply(x=w1128, y=w1127) -> (x*y=w1126:dbl)
          n690 = Multiply(x="2D Motion Frequency (Hz)", y=w1126) -> (x*y=w1102:dbl)
          n691 = Subtract(x=1.5707963267948966, y=w1117) -> (x-y=w1103:dbl)
          n692 = Subtract(x=w1102, y=1.5707963267948966) -> (x-y=w1124:dbl)
          n693 = Add(x=w1102, y=w1103) -> (x+y=w1104:dbl)
          n694 = Cosine(x=w1124) -> (cos(x)=w1123:dbl)
          n695 = Sine(x=w1124) -> (sin(x)=w1122:dbl)
          n696 = Multiply(x=w1123, y=w1119) -> (x*y=w1112:dbl)
          n697 = Cosine(x=w1104) -> (cos(x)=w1121:dbl)
          n698 = Sine(x=w1104) -> (sin(x)=w1120:dbl)
          n699 = Multiply(x=w1122, y=w1119) -> (x*y=w1111:dbl)
          n700 = Multiply(x=w1121, y=w1119) -> (x*y=w1116:dbl)
          n701 = Multiply(x=w1120, y=w1119) -> (x*y=w1113:dbl)
          n702 = Add(x=w1112, y=w1110) -> (x+y=w1099:dbl)
          n703 = Add(x=w1111, y=w1109) -> (x+y=w1097:dbl)
          n704 = Add(x=w1116, y=w1115) -> (x+y=w1101:dbl)
          n705 = Add(x=w1113, y=w1114) -> (x+y=w1100:dbl)
          n706 = property on="BD 1 Frequency 1 (MHz)" class="DigNum (strict)"("Val(Sgnl)"=w1099) -> ()  [unwired: 2 in, 2 out]
          n707 = property on="BD 2 Frequency 1 (MHz)" class="DigNum (strict)"("Val(Sgnl)"=w1097) -> ()  [unwired: 2 in, 2 out]
          n708 = property on="BD 1 Frequency 2 (MHz)" class="DigNum (strict)"("Val(Sgnl)"=w1101) -> ()  [unwired: 2 in, 2 out]
          n709 = property on="BD 2 Frequency 2 (MHz)" class="DigNum (strict)"("Val(Sgnl)"=w1100) -> ()  [unwired: 2 in, 2 out]
          n710 = Build Array (concatenate)(w1098, w1099) -> (w1095:dbl[])
          n711 = Build Array (concatenate)(w1096, w1097) -> (w1094:dbl[])
          n712 = local read "Stop All"() -> (w1106:bool)
          n713 = Bundle(w1095, w1094) -> (→"XY Graph":cluster{dbl[], dbl[]})  [unwired: 1 in]
          n714 = Or(x=w1106, y="Stop Moving") -> (x .or. y?=w1107:bool)
          n715 = node-c288() -> ()  [unwired: 1 in, 1 out]
        }
        n716 = node-c288(w1091) -> ()  [unwired: 1 out]
      }
      event "Stop All": Value Change {
        # "Stopping blue laser before shutting off program"
        n717 = event-data() -> ()  [unwired: 1 in, 5 out]
        n718 = local read "Delay (ms)"() -> (w1138:i32)
        n719 = call "serial write macro.vi"("String"="l0", "Delay (ms)"=w1138, "VISA resource name"=w1141) -> ("read buffer"=w1136:string, "error out"=w1137:errorcluster, "VISA resource name out"=w1140:refnum<visa-resource-name>)
        n720 = local write "read blue buffer"(w1136) -> ()
        n721 = local write "Blue Error Out"(w1137) -> ()
        n722 = VISA Close(VISA resource name=w1140) -> ()  [unwired: 1 in, 1 out]
        n723 = local read "Stop All"() -> (w1142:bool)
      }
    }
    n724 = node-c288() -> ()  [unwired: 1 in, 1 out]
  }
  n725 = node-c288() -> (w17:T23)  [unwired: 4 out]
  n726 = node-c288(3 ("Processor")) -> (w131:T23)  [unwired: 3 out]
  n727 = node-c288(2 ("Processor")) -> (w133:T23)  [unwired: 3 out]
  n728 = node-c288() -> (w135:T23)  [unwired: 4 out]
  n729 = node-c288(i64 1 ("Period"), 1 ("Processor")) -> (w206:T23)  [unwired: 2 out]
  n730 = while "Duncan's play event loop" {
    stop <- w1144 stop-if-true
    n731 = Create User Event(user event datatype=TRUE ("Boolean")) -> (user event=w1145:refnum<user-event>)  [unwired: 1 in, 1 out]
    n732 = Create User Event(user event datatype=TRUE ("Boolean")) -> (user event=w1152:refnum<user-event>)  [unwired: 1 in, 1 out]
    n733 = global write "Global for fluorescence simulation mean (30 samples), (power series).vi" "Red Signal"(w1145) -> ()
    n734 = global write "Global for fluorescence simulation mean (30 samples), (power series).vi" "Green Signal"(w1152) -> ()
    n735 = register-events(w1152, w1145) -> (reference out=w1151:refnum<event-registration>)  [unwired: 2 in, 1 out]
    n736 = event shown="[1] \"Get Fluorophore\": Value Change" {
      selector: w1151 -> [_ _ _ _]
      dyn-events: _ -> [_ _ _ _]
      timeout: 100 -> [_ _ _ _]
      event Timeout {
        n737 = event-data() -> ()  [unwired: 1 in, 2 out]
      }
      event "Get Fluorophore": Value Change {
        n738 = event-data() -> ("OldVal"=w1154:bool)  [unwired: 1 in, 4 out]
        n739 = case shown="True" w1154 {
          selector: w1154 -> [_ w1155]
          frame False {
          }
          frame True {
            n740 = property on="Move to Position 3" class="Bool"("Val(Sgnl)"=w1155) -> ()  [unwired: 2 in, 2 out]
            n741 = case shown="1" "Numeric" {
              frame 0, Default {
              }
              frame 1 {
                n742 = property on="Green Laser ON" class="Bool (strict)"("Val(Sgnl)"=TRUE ("Value (Signaling)")) -> ()  [unwired: 2 in, 2 out]
              }
              frame 2 {
                n743 = property on="Red Laser ON" class="Bool (strict)"("Val(Sgnl)"=TRUE) -> ()  [unwired: 2 in, 2 out]
              }
            }
          }
        }
      }
      event User Event {
        n744 = event-data() -> ("Boolean"=w1159:bool)  [unwired: 1 in, 3 out]
        "Green Fluorophore" <- w1159
        n745 = property on="Get Fluorophore" class="Bool (strict)"("Val(Sgnl)"=w1159) -> ()  [unwired: 2 in, 2 out]
      }
      event User Event {
        n746 = event-data() -> ("Boolean"=w1160:bool)  [unwired: 1 in, 3 out]
        "Red Fluorophore" <- w1160
        n747 = property on="Get Fluorophore" class="Bool (strict)"("Val(Sgnl)"=w1160) -> ()  [unwired: 2 in, 2 out]
      }
    }
    n748 = property on="Get Fluorophore" class="Bool (strict)"("Val(Sgnl)"="Get Fluorophore") -> ()  [unwired: 2 in, 2 out]
    n749 = Wait (ms)(milliseconds to wait=u32 100) -> ()  [unwired: 1 out]
    n750 = local read "Stop All"() -> (w1143:bool)
    n751 = Or(x=w1143, y="stop") -> (x .or. y?=w1144:bool)
  }
  n752 = timed-loop "Rough control of MCL mirror stage (debugging)" {
    tunnel: w23 -> [w1163]
    tunnel: [w1162] -> w261
    timing: w17 -> [_]
    timing-out: [_] -> w16
    stop <- w1162 stop-if-true
    n753 = node-c288() -> ()  [unwired: 2 out]
    n754 = case shown="1" "MCL Mode" {
      tunnel: w1163 -> [_ w1166 w1213]
      frame 0, Default {
      }
      frame 1 {
        n755 = node-c288() -> (w1168:T23)  [unwired: 4 out]
        n756 = timed-loop "Oscillate MCL mirror" {
          timing: w1168 -> [_]
          timing-out: [_] -> w1167
          tunnel: w1166 -> [w1207]
          i -> [w1206]
          stop <- w1169 stop-if-true
          n757 = node-c288() -> (w1205:i64)  [unwired: 1 out]
          n758 = Multiply(x="AO1", y=32767.0) -> (x*y=w1201:dbl)
          n759 = Multiply(x="AO2", y=32767.0) -> (x*y=w1196:dbl)
          n760 = Divide(x=w1201, y=10.0) -> (x/y=w1202:dbl)
          n761 = Divide(x=w1196, y=10.0) -> (x/y=w1197:dbl)
          n762 = To Word Integer(number=w1202) -> (16bit integer=w1194:i16)
          n763 = To Word Integer(number=w1197) -> (16bit integer=w1193:i16)
          n764 = Divide(x=w1205, y=i64 1000) -> (x/y=w1176:dbl)
          n765 = Multiply(x=w1176, y=w1206) -> (x*y=w1187:dbl)
          n766 = Multiply(x="Osc. freq. (Hz) 2", y=6.283185307179586) -> (x*y=w1188:dbl)
          n767 = Multiply(x=w1188, y=w1187) -> (x*y=w1186:dbl)
          n768 = Sine(x=w1186) -> (sin(x)=w1185:dbl)
          n769 = Multiply(x=w1185, y="Osc. amp. (V)") -> (x*y=w1183:dbl)
          n770 = Add(x=w1183, y="Osc. center (V)") -> (x+y=w1181:dbl)
          n771 = Divide(x=w1181, y=10.0) -> (x/y=w1179:dbl)
          n772 = Multiply(x=w1179, y=32767.0) -> (x*y=w1174:dbl)
          n773 = Select(t=w1174, s="Scan axis", f=w1194) -> (s? t:f=w1192:dbl)
          n774 = Select(t=w1193, s="Scan axis", f=w1174) -> (s? t:f=w1191:dbl)
          n775 = local read "MCL Mode"() -> (w1173:u16)
          n776 = Not Equal?(x=w1173, y=u16 1) -> (x != y?=w1170:bool)
          n777 = local read "Stop All"() -> (w1171:bool)
          n778 = xnode "Read/Write Control"("FPGA VI Reference In"=w1207, "AO1"=w1192, "AO2"=w1191) -> ()  [unwired: 1 in, 2 out]
          n779 = Compound Arithmetic op=OR(w1171, w1170) -> (w1169:bool)
          n780 = node-c288() -> ()  [unwired: 2 out]
        }
        n781 = node-c288(w1167) -> ()  [unwired: 1 out]
      }
      frame 2 {
        n782 = case shown="True" "Start Scan" {
          tunnel: w1213 -> [_ w1225]
          frame False {
          }
          frame True {
            n783 = Subtract(x="End (V)", y="Begin (V)") -> (x-y=w1221:dbl)
            n784 = Decrement(x="N Points") -> (x-1=w1220:dbl)
            n785 = Divide(x=w1221, y=w1220) -> (x/y=w1218:dbl)
            n786 = for {
              N: "N Points" -> [_]
              tunnel: "Begin (V)" -> [w1238]
              tunnel: w1225 -> [w1230]
              tunnel: [w1229] -> w1224 mode=indexing
              tunnel: w1218 -> [w1228]
              tunnel: [w1226] -> w1217 mode=indexing
              i -> [w1237]
              n787 = Multiply(x=w1228, y=w1237) -> (x*y=w1236:dbl)
              n788 = Add(x=w1238, y=w1236) -> (x+y=w1233:dbl)
              n789 = local read "Scan axis"() -> (w1227:bool)
              n790 = local read "AO1"() -> (w1235:dbl)
              n791 = local read "AO2"() -> (w1234:dbl)
              n792 = Select(t=w1233, s=w1227, f=w1235) -> (s? t:f=w1232:dbl)
              n793 = Select(t=w1234, s=w1227, f=w1233) -> (s? t:f=w1231:dbl)
              n794 = flat-sequence {
                tunnel: w1232 -> [w1242]
                tunnel: w1231 -> [w1241]
                tunnel: w1230 -> [w1239]
                tunnel: [w1252] -> w1229
                tunnel: [w1251] -> w1226
                frame #0 {
                  w1245 = 10.0 ("y")
                  w1240 = 32767.0 ("y")
                  n795 = Multiply(x=w1242, y=w1240) -> (x*y=w1248:dbl)
                  n796 = Multiply(x=w1241, y=w1240) -> (x*y=w1246:dbl)
                  n797 = Divide(x=w1248, y=w1245) -> (x/y=w1249:dbl)
                  n798 = Divide(x=w1246, y=w1245) -> (x/y=w1247:dbl)
                  n799 = To Word Integer(number=w1249) -> (16bit integer=w1243:i16)
                  n800 = To Word Integer(number=w1247) -> (16bit integer=w1244:i16)
                  n801 = xnode "Read/Write Control"("FPGA VI Reference In"=w1239, "AO1"=w1243, "AO2"=w1244) -> ()  [unwired: 1 in, 2 out]
                }
                frame #1 {
                  n802 = Wait (ms)(milliseconds to wait="DAQ Delay (ms)") -> ()  [unwired: 1 out]
                }
                frame #2 {
                  n803 = local read "Slow mean"() -> (w1252:dbl)
                  n804 = local read "Sigma"() -> (w1251:dbl)
                }
              }
            }
            n805 = Bundle("Begin (V)"="Begin (V)", w1218, w1224) -> (→"MCL Scan":cluster{"Begin (V)":dbl, dbl, dbl[]})  [unwired: 1 out]
            n806 = Bundle("Begin (V)"="Begin (V)", w1218, w1217) -> (→"MCL Scan 2":cluster{"Begin (V)":dbl, dbl, dbl[]})  [unwired: 1 out]
          }
        }
      }
    }
    n807 = local read "Stop All"() -> (w1162:bool)
    n808 = node-c288() -> ()  [unwired: 2 out]
  }
  n809 = timed-loop "Oscillate Trap/AOM (fishing, conjugate plane alignment)" {
    tunnel: w23 -> [w1254]
    tunnel: [w1253] -> w136
    timing: w131 -> [_]
    timing-out: [_] -> w130
    stop <- w1253 stop-if-true
    n810 = node-c288() -> ()  [unwired: 2 out]
    n811 = event shown="[0] \"Oscillate Set 1\", \"Fish for Tether\": Value Change" {
      selector: _ -> [_ _ _]
      dyn-events: _ -> [_ _ _]
      timeout: _ -> [_ _ _]
      tunnel: w1254 -> [w1261 _ _]
      tunnel: [FALSE ("Stop All") _ w1859] -> w1253
      event "Oscillate Set 1", "Fish for Tether": Value Change {
        n812 = event-data() -> ()  [unwired: 6 out]
        n813 = local read "Oscillate Set 1"() -> (w1260:bool)
        n814 = Or(x=w1260, y="Fish for Tether") -> (x .or. y?=w1258:bool)